vi "UHR-Fleezers Control (host) - Avogadro v1.vi"() -> ()   [LabVIEW 2014] (continued)
2.430581438642532, 2.430926786095764, 2.431356364635146, 2.4317856379894374, 2.4321182287057037, 2.432515152439944, 2.4328666951506044, 2.4333012482070333, 2.433380260628069, 2.4336372264778565, 2.433614551225319, 2.4335650502029416, 2.4334475234229562, 2.4333011261329975, 2.433007934812456, 2.432660908841205, 2.4323364970854775, 2.431945677053128, 2.4314603106784243, 2.4310055848872327, 2.4304504226813495, 2.429832483901481, 2.4295840632343437, 2.430289254432808, 2.430990173039951, 2.431600177007347, 2.4321969969786634, 2.4325847651600614, 2.432949278237247, 2.4332937711722127, 2.4336035035248855, 2.4338471633045415, 2.43411856440931, 2.4341327249977085, 2.434035584582046, 2.433841761528369, 2.4335344706564492, 2.4331067537461406, 2.4326152531510337, 2.4322612994781294, 2.4318525650807197, 2.4314216742454273, 2.431016113773001, 2.4305053865169173, 2.4301109347819363, 2.4296082033753423, 2.4291993469038955, 2.4287146214178863, 2.428318033387242, 2.427947843867298, 2.427710409863576, 2.4275749382000127, 2.427406750694291, 2.4272803430280403, 2.427055726798301, 2.4267129123813582, 2.426466566972866, 2.4265800653096097, 2.4264022339548923, 2.42636317026276, 2.4261367534409617, 2.4259769585253403, 2.4209620349742065, 2.420926541947684, 2.420983275856805, 2.4211451155125534, 2.4212160100100664, 2.421280648213139, 2.4213176976836435, 2.421396557512131, 2.4214452955717625, 2.4213891109958166, 2.4212491836298677, 2.42129685354167, 2.4214397106845302, 2.4216707358012615, 2.421910672322762, 2.422093997009182, 2.422323526718951, 2.422714682454901, 2.4230255439924244, 2.4235496993926793, 2.423987121189, 2.4243907895138364, 2.424590746787921, 2.4248405102694734, 2.4251454512161543, 2.425395336771748, 2.4256246223334412, 2.4256791894283816, 2.4256945402386467, 2.4256017639698415, 2.4255321207312166, 2.4253109836115545, 2.4250167851802042, 2.4246725974303374, 2.42415070039979, 2.423467665639209, 2.4229174169133496, 2.422391308328497, 2.4217404095583976, 2.4211572618793236, 2.4211068453016704, 2.421682821131013, 2.4222059999389587, 2.4226697897274634, 2.423094027527689, 2.4236765037995527, 2.4239891048921156, 2.424316080202641, 2.4245177770317685, 2.424673329874565, 2.424790337839895, 2.424709433271276, 2.4246918851283272, 2.424496749778738, 2.424243598742637, 2.4239404889065184, 2.423611957152008, 2.423288918729205, 2.4229048432874487, 2.422400921658983, 2.421536027100433, 2.421068910794393, 2.42072060304574, 2.4203089999084413, 2.420026642658768, 2.4196926480910648, 2.4193796807763888, 2.4190245674001263, 2.418800988799702, 2.418650532547986, 2.418678823206272, 2.4186175725577495, 2.4184317148350396, 2.418353709524823, 2.418170720542003, 2.418003967406226, 2.417792291024499, 2.4176316110721063, 2.4175349894711093, 2.4173629566331947, 2.417207373271886, 2.41730030213324, 2.4174544816431127, 2.4175632801293956, 2.417742790002129, 2.4180165410321286, 2.418110812707902, 2.4181535996581878, 2.418099612414924, 2.418115939817495, 2.417978545487829, 2.418120883816028, 2.4182416150395163, 2.4184165471358328, 2.418608569597455, 2.418898007141329, 2.419110782189396, 2.4194311349833684, 2.4197565538499073, 2.4202420422986477, 2.420669942320011, 2.4211170995208566, 2.4214806360057346, 2.4217368999297992, 2.422168858912926, 2.42250303659169, 2.4226787316507403, 2.422940610980556, 2.4229851069673676, 2.423065034943685, 2.423195989867848, 2.423032593768114, 2.4228180791650056, 2.422440992461923, 2.422032990508745, 2.421433820612196, 2.4209468062379784, 2.420461653492839, 2.4199261757255752, 2.4194091616565454, 2.419384411145355, 2.420076479384742, 2.420686025574504, 2.4213249000518786, 2.4217745902890058, 2.4222578508865595, 2.4227300332651676, 2.423039735099329, 2.4233286843470467, 2.423545365764331, 2.4236784875026656, 2.4237635120700705, 2.423771416364023, 2.4236595660267928, 2.423627063814199, 2.423647724845113, 2.4233858149967897, 2.4231237220374098, 2.4228541520432048, 2.4225346842860156, 2.4221234473708244, 2.42164976958525, 2.4213015839106395, 2.420928800317386, 2.420634083071378, 2.4201690725424907, 2.4198965422528707, 2.4196620685445707, 2.4194428540910047, 2.4193014923551144, 2.419234412671285, 2.419066042054504, 2.418075472273929, 2.4178200628681212, 2.417850154118468, 2.418008453627117, 2.4178781701101624, 2.4178394421216405, 2.417761833552041, 2.4177437055574154, 2.406593401898251, 2.4039209265419417, 2.4035707571642124, 2.4033807489242163, 2.4033286843470503, 2.403229651783802, 2.4031948301644883, 2.4032014831995547, 2.4031528366954533, 2.4030944242683163, 2.4030547196874847, 2.4031530808435244, 2.4033223975341, 2.40348313852351, 2.40359135715811, 2.403636158330024, 2.4037828302865623, 2.4041361735892806, 2.404406811731312, 2.4048561662648353, 2.405317697683637, 2.4055910214545078, 2.405806115909293, 2.406070070497755, 2.4062391125217393, 2.4064092226935587, 2.406426221503337, 2.4066071047090016, 2.4065373393963383, 2.4063661610766838, 2.4061467940305765, 2.4056369518112697, 2.405410107730332, 2.4051367839594686, 2.4046134830774855, 2.404083742789998, 2.4035795159764346, 2.4029824823755557, 2.402330027161473, 2.4015955992309306, 2.401533219397561, 2.4021967223120804, 2.402693655201877, 2.4032305063020662, 2.4036669820245944, 2.4041217383342954, 2.4044415417950957, 2.4046650288399882, 2.4048795434430934, 2.404969725638594, 2.4047648243659756, 2.4047524948881476, 2.404638966032896, 2.40437504196295, 2.40416742454298, 2.404013458662675, 2.4035543076876085, 2.4030866725669062, 2.40267934202093, 2.402205328531752, 2.401525803399758, 2.400994109927664, 2.4005073702200335, 2.4000125431073918, 2.399666432691425, 2.399542344431894, 2.3991321756645387, 2.398807275612653, 2.3985068819238817, 2.398275582140563, 2.398063081759082, 2.3979806817834977, 2.3978454847865187, 2.397760826441233, 2.397697225867489, 2.397577776421397, 2.3974082461012607, 2.3973235572374643, 2.3971585741752346, 2.3969482100894144, 2.399339609973449, 2.3996950895718228, 2.3997654957731838, 2.3997879573961587, 2.3999571214941846, 2.4000226142155188, 2.4000767235328184, 2.40004583880123, 2.4001323587755943, 2.4002205877864884, 2.400232245857111, 2.4004011047700407, 2.4005788750877337, 2.400797845393222, 2.401105594042782, 2.4016392406994806, 2.4019311502426213, 2.4022950529496114, 2.4027085787530114, 2.4032281868953476, 2.4037702871791677, 2.4041618091372414, 2.404428052613911, 2.404843684194461, 2.4051377300332626, 2.4055124362926077, 2.4056537064729686, 2.405908444471569, 2.4058568071535325, 2.4058369701223734, 2.4055328836939545, 2.4053381756035, 2.4050690023499244, 2.404632801293984, 2.4042121951963833, 2.4037009796441504, 2.4032916043580337, 2.4027538987395824, 2.4021463362529354, 2.401571764275031, 2.4014757225257117, 2.4020927152317855, 2.4026458632160357, 2.4031801507614308, 2.4036126590777247, 2.4041590929898926, 2.404629566331979, 2.4050496536149155, 2.4053699758903715, 2.405671163060388, 2.4060234687337823, 2.40607593005157, 2.4060553910946934, 2.4060759910885916, 2.4059835200048774, 2.405767418439276, 2.4055522934659828, 2.405272835474708, 2.4049551377910685, 2.4046062196722304, 2.403999328592787, 2.4035610522782016, 2.4032514419995685, 2.40294955290383, 2.4027128513443357, 2.402457594531081, 2.4022258674886334, 2.402022461622973, 2.4018425855281196, 2.401701437421794, 2.401658528397469, 2.4015787224951906, 2.401492141483804, 2.401444593646041, 2.4014353160191626, 2.401671651356542, 2.4017135837885633, 2.4018295846430813, 2.401837549974056, 2.4017239906002943, 2.424597918637651, 2.4246118350779726, 2.424565507980587, 2.42459965819269, 2.424594073305456, 2.4245285195471036, 2.4245402691732525, 2.4247233802301023, 2.424646931363866, 2.424751487777332, 2.4247339396343883, 2.424781212805563, 2.424835016937768, 2.4247366557817274, 2.4247208777123284, 2.424638264107179, 2.424499588000122, 2.4244687337870374, 2.424328531754507, 2.42422482985931, 2.4241373943296605, 2.424011902218693, 2.4236910306100627, 2.42360475478377, 2.4235302896206514, 2.4235555894650047, 2.4235575731681207, 2.4235125888851528, 2.42349827570421, 2.4234156010620382, 2.4232872707296917, 2.4231805169835416, 2.4231496932889733, 2.4230475478377596, 2.422977690969568, 2.4230106204412944, 2.4229536423841003, 2.4229382305368117, 2.422888180181274, 2.422950346385075, 2.4229270302438395, 2.4229190649128642, 2.4226663716544024, 2.4226755882442625, 2.422584673604535, 2.422560686056087, 2.4226352732932437, 2.4229356364635053, 2.4229169286171994, 2.4229865108188076, 2.424675008392584, 2.4252596514786156, 2.425283150730913, 2.4254429456465294, 2.4254956511123926, 2.425613177892387, 2.4259598071230144, 2.4260010681478272, 2.4260692770165075, 2.426234687337868, 2.4262993865779587, 2.4264269844660737, 2.426569872127441, 2.426780083620717, 2.4270130008850312, 2.427282967619854, 2.4273390301217663, 2.4276983855708405, 2.42808078249458, 2.4286301461836577, 2.4290816675313547, 2.4294141056550753, 2.4298842738120636, 2.430225898007133, 2.430553727835928, 2.4309037141026, 2.431134952848902, 2.431286141544846, 2.431253883480331, 2.431170751060514, 2.4310626850184627, 2.430942991424295, 2.430730918301947, 2.4304457228308918, 2.430165593432409, 2.4297568285164917, 2.4296153447065603, 2.4291805169835476, 2.428557847834706, 2.4280869472334916, 2.4281168858912854, 2.4287542954802084, 2.4295111545152106, 2.4301620838038196, 2.4307819147312806, 2.4313480025635523, 2.4315205542161324, 2.4318085879085625, 2.4321279335917176, 2.4323574938199934, 2.4325492721335404, 2.432612842188781, 2.432604907376317, 2.432455244605846, 2.432274117252107, 2.4319997863704295, 2.431997924741351, 2.431658742027037, 2.4312776573992108, 2.43085882137516, 2.4304665974913706, 2.429956236457407, 2.4296554155095036, 2.4292895596179056, 2.4290475478377633, 2.4287481612598, 2.428205755790881, 2.427885982848589, 2.4276909695730398, 2.4276541337320996, 2.4274905850398176, 2.4276107974486476, 2.4276034424878614, 2.4273903622547013, 2.427224982451853, 2.4271848200933808, 2.4269551988280877, 2.4267975402081343, 2.4267496261482577, 2.426536301767019, 2.402900875881221, 2.4031380657368633, 2.403752037110504, 2.4042728659932218, 2.4050129093295034, 2.4052575457014633, 2.4056152226325183, 2.405845484786517, 2.405950468459114, 2.405743491927848, 2.4051299783318587, 2.404316751609847, 2.404051820429085, 2.404275246436962, 2.404634113589891, 2.4047569811090383, 2.4051246070741885, 2.4055120090334725, 2.4058326670125365, 2.4063693044831678, 2.4067348857081807, 2.406775078585158, 2.4071752067628993, 2.407703695791494, 2.4078374584185243, 2.4081329691457833, 2.408269081698046, 2.408250526444283, 2.4082946256904774, 2.408282418286684, 2.4080811792351993, 2.4081080355235382, 2.4079442732016916, 2.407491012298956, 2.4070355235450283, 2.4066586809900175, 2.4060685750907864, 2.4054919278542384, 2.4049438764610716, 2.4042894070253564, 2.4041783196508693, 2.404856166264839, 2.405279549546793, 2.4057430646687172, 2.4062998138370912, 2.4066878872035886, 2.4067595446638355, 2.4071760307626544, 2.4073634144108387, 2.4075584582048983, 2.4076643879512893, 2.4077086703085353, 2.407621631519512, 2.4074461195715173, 2.4071774346140895, 2.4067588427381175, 2.4066013977477314, 2.406143955809193, 2.405616870632034, 2.4051503952146938, 2.4046809900204456, 2.4041257972960577, 2.4037431867427563, 2.403418012024289, 2.4030837122714876, 2.402824457533492, 2.4025822931608016, 2.4023588061159042, 2.402216620380259, 2.4021348612933697, 2.401934965056304, 2.401611224707785, 2.4014654683065273, 2.401353160191649, 2.40129486983855, 2.4013071077608505, 2.4011179235206104, 2.4010649128696504, 2.400908413953057, 2.400771691030605, 2.4020871303445483, 2.4011822260200764, 2.4007248451185617, 2.4004102298043732, 2.3998872951445063, 2.399638630329293, 2.3994718771935144, 2.399311044648575, 2.39913538010803, 2.399068422498242, 2.398960966826375, 2.3986503494369287, 2.3986418958098024, 2.398676351207001, 2.3988180181279932, 2.398978362376777, 2.3994265877254564, 2.3998741111484096, 2.4001463972899555, 2.4005340433973146, 2.4009977416302934, 2.401073030793167, 2.4014315622424993, 2.401741813409832, 2.40197305215613, 2.4023876766258674, 2.4026499526963048, 2.402819330423898, 2.402831354716631, 2.4027815790276805, 2.402703329569381, 2.4028177129428956, 2.4025652333140015, 2.402136692403945, 2.40164436780907, 2.400992217780078, 2.4004347361674796, 2.4000155034028174, 2.3995320902127117, 2.3990206610309106, 2.3991094698934887, 2.3998409070100983, 2.400514847254854, 2.4011603442487814, 2.401726035340429, 2.4021230506302067, 2.402113071077605, 2.4025136875514983, 2.4026888027588678, 2.4028879665517118, 2.4027249366740917, 2.4025446333201073, 2.402652150028987, 2.402734397412022, 2.402406781212803, 2.402132328257089, 2.4022540971098962, 2.4020598773155912, 2.40171459089938, 2.401353556932273, 2.4009453413495225, 2.400347270119321, 2.400007446516312, 2.399501022370065, 2.3991158482619657, 2.39877190466017, 2.398409833063749, 2.3981063264870137, 2.3978381298257374, 2.397473036896876, 2.3972162541581454, 2.396722952970971, 2.3964001892147513, 2.3962673421430067, 2.3961395306253186, 2.396097903378391, 2.39589822077089, 2.3957543565172243, 2.3955935239722863, 2.3953248084963525, 2.3711730704672336, 2.3691772515030287, 2.368657460249641, 2.368525070955532, 2.368504135258033, 2.3685816522720984, 2.369277321695607, 2.369537125766776, 2.3694836878566834, 2.3696178167058295, 2.3696047242652627, 2.3696505325479884, 2.369786339915157, 2.369958159123507, 2.3701187780388797, 2.3703828547013766, 2.3703139744254886, 2.3705926999725313, 2.3709521469771375, 2.371376079592269, 2.371703726310003, 2.372084261604661, 2.372402600177005, 2.3726291390728416, 2.372854182561725, 2.3730838648640367, 2.3734214300973506, 2.3735248878444755, 2.373402447584457, 2.3732737815485083, 2.373095217749563, 2.3729121982482355, 2.3726266060365604, 2.372233710745564, 2.371795739616075, 2.371224280526134, 2.370653157139803, 2.3700431836909024, 2.369352122562329, 2.3686639912106693, 2.368520035401466, 2.3687518234809373, 2.3692865382854666, 2.369742362743001, 2.3701869258705393, 2.370600848414558, 2.370890102847375, 2.371232123783071, 2.3714059266945355, 2.371503616443369, 2.3714757835627265, 2.371450148014769, 2.371331064790795, 2.371147282326728, 2.3709205603198336, 2.370594347972041, 2.3701680654316837, 2.369824732200076, 2.369418927579573, 2.369010559404277, 2.368637379070405, 2.3684136173589247, 2.368100344859156, 2.367791741691333, 2.367505630664996, 2.36728153324991, 2.3670190130314013, 2.3668691671498707, 2.366697531052578, 2.36665858943449, 2.3665348979155816, 2.3662927030243854, 2.366204962309637, 2.366202612384408, 2.3661817987609473, 2.3661056550798043, 2.3660763878292177, 2.366077394940028, 2.3660827051606765, 2.36617389446699] caption="Most Recent Time Trace"
  out "Values":dbl[](array[numeric])=[-0.06760925671124465, 0.04910653407946759, 4.445727607043673, -0.09151692288622436, 0.04947272910700923, 3.2662948698385565, -0.09383489136567569, 3.086667088839382, -0.1922671172735984, 2.235330652790918, -0.05378544658904728, -0.006441883611510604, 2.422861781670583]
  out "All Signals":waveform(dbl)[](graph)=[{"t0"=timestamp(302.5999999999914 s since 1904-01-01), "dt"=0.15, "Y"=[0.0], "attributes"=variant("NI_ChannelName"=variant(string "APD 1"))}, {"t0"=timestamp(302.5999999999914 s since 1904-01-01), "dt"=0.15, "Y"=[0.0], "attributes"=variant("NI_ChannelName"=variant(string "APD 2"))}, {"t0"=timestamp(302.5999999999914 s since 1904-01-01), "dt"=0.15, "Y"=[0.0], "attributes"=variant("NI_ChannelName"=variant(string "APD 3"))}, {"t0"=timestamp(302.5999999999914 s since 1904-01-01), "dt"=0.1, "Y"=[-0.06757372680085764, -0.06764478662163165], "attributes"=variant("NI_ChannelName"=variant(string "T1 Y"))}, {"t0"=timestamp(302.5999999999914 s since 1904-01-01), "dt"=0.1, "Y"=[0.049145059705078195, 0.0490680084538571], "attributes"=variant("NI_ChannelName"=variant(string "T1 X"))}, {"t0"=timestamp(302.5999999999914 s since 1904-01-01), "dt"=0.1, "Y"=[4.445783654286312, 4.445671559801015], "attributes"=variant("NI_ChannelName"=variant(string "T1 Sum"))}, {"t0"=timestamp(302.5999999999914 s since 1904-01-01), "dt"=0.1, "Y"=[-0.09151746422952804, -0.09151638154292077], "attributes"=variant("NI_ChannelName"=variant(string "T2 Y"))}, {"t0"=timestamp(302.5999999999914 s since 1904-01-01), "dt"=0.1, "Y"=[0.04952704956149684, 0.04941840865252152], "attributes"=variant("NI_ChannelName"=variant(string "T2 X"))}, {"t0"=timestamp(302.5999999999914 s since 1904-01-01), "dt"=0.1, "Y"=[3.266107669301433, 3.2664820703756816], "attributes"=variant("NI_ChannelName"=variant(string "T2 Sum"))}, {"t0"=timestamp(302.5999999999914 s since 1904-01-01), "dt"=0.1, "Y"=[-0.09387435236185547, -0.0937954303694959], "attributes"=variant("NI_ChannelName"=variant(string "T1 FB X"))}, {"t0"=timestamp(302.5999999999914 s since 1904-01-01), "dt"=0.1, "Y"=[3.0867849971007453, 3.0865491805780243], "attributes"=variant("NI_ChannelName"=variant(string "T1 FB Sum"))}, {"t0"=timestamp(302.5999999999914 s since 1904-01-01), "dt"=0.1, "Y"=[-0.192305278199375, -0.19222895634782178], "attributes"=variant("NI_ChannelName"=variant(string "T2 FB X"))}, {"t0"=timestamp(302.5999999999914 s since 1904-01-01), "dt"=0.1, "Y"=[2.2353390301217684, 2.235322275460067], "attributes"=variant("NI_ChannelName"=variant(string "T2 FB Sum"))}, {"t0"=timestamp(302.5999999999914 s since 1904-01-01), "dt"=0.1, "Y"=[-0.053826675533845625, -0.05374421764424899], "attributes"=variant("NI_ChannelName"=variant(string "T3 Y/ PSD Y"))}, {"t0"=timestamp(302.5999999999914 s since 1904-01-01), "dt"=0.1, "Y"=[-0.006535476968530134, -0.006348290254491073], "attributes"=variant("NI_ChannelName"=variant(string "T3 X / PSD X"))}, {"t0"=timestamp(302.5999999999914 s since 1904-01-01), "dt"=0.1, "Y"=[2.422819391460915, 2.422904171880237], "attributes"=variant("NI_ChannelName"=variant(string "T3 Sum / PSD sum"))}]
  in  "Signals to Plot":i32(listbox)=18
  out "Trap Disp. Freq. (Hz)":dbl=10.0 caption="Freq. (Hz)" format="%#_6p"
  out "Display Period (s)":dbl=0.1 caption="Period (s)" format="%#_6p"
  in  "Trap Disp. Downsample":dbl=10000.0 caption="Downsample" max=20000.0
  in  "APD Disp. Scale":dbl=0.1 caption="Scale (Divide,\nfor above plot only)"
  in  "APD Disp. Downsample":dbl=150.0 caption="Integrate" max=200.0
  out "APD Display Freq. (Hz)":dbl=6.666666666666667 caption="Freq. (Hz)"
  out "APD Display Period (s)":dbl=0.15 caption="Period (s)"
  out "FFT 1":cluster{"f0":dbl, "df":dbl, "magnitude":dbl[]}[](graph)=[{"f0"=0.0, "df"=3.3333333333333335, "magnitude"=array[10000 elements]}, {"f0"=0.0, "df"=3.3333333333333335, "magnitude"=array[10000 elements]}]
  out "FFT 2":cluster{"f0":dbl, "df":dbl, "magnitude":dbl[]}[](graph)
  in  "FFT 1 Choice 1":u16(ring) items=["T1 Y", "T1 X", "T1 Sum", "T2 Y", "T2 X", "T2 Sum", "T1 FB X", "T1 FB Sum", "T2 FB X", "T2 FB Sum", "PSD Y", "PSD X", "PSD Y Sum", "none"]
  in  "FFT 2 Choice 1":u16(ring)=13 items=["T1 Y", "T1 X", "T1 Sum", "T2 Y", "T2 X", "T2 Sum", "T1 FB X", "T1 FB Sum", "T2 FB X", "T2 FB Sum", "PSD Y", "PSD X", "PSD Y Sum", "none"]
  in  "FFT 1 Choice 2":u16(ring)=1 items=["T1 Y", "T1 X", "T1 Sum", "T2 Y", "T2 X", "T2 Sum", "T1 FB X", "T1 FB Sum", "T2 FB X", "T2 FB Sum", "PSD Y", "PSD X", "PSD Y Sum", "none"]
  in  "FFT 2 Choice 2":u16(ring)=13 items=["T1 Y", "T1 X", "T1 Sum", "T2 Y", "T2 X", "T2 Sum", "T1 FB X", "T1 FB Sum", "T2 FB X", "T2 FB Sum", "PSD Y", "PSD X", "PSD Y Sum", "none"]
  in  "Compute FFT":bool
  in  "Reset FFT":bool
  in  "# Spectra to Ave.":dbl=25.0
  out "Ave. Time (s)":dbl=7.5
  out "1 Channel":waveform(dbl)(graph)={"t0"=timestamp(0 s since 1904-01-01), "dt"=1e-05, "Y"=array[20000 elements], "attributes"=variant("NI_ChannelName"=variant(string "T1 X"))}
  out "Slow mean":dbl=0.04910653407946759 format="%0.2f"
  in  "Slow mean N ave.":dbl=1.0 min=1.0 step=1.0
  out "Mean Intensity":dbl=0.049106534079467676
  out "Sigma":dbl=0.00020183735235839546
  out "Sigma/Mean":dbl=0.004110193401793903
  in  "Subtract mean":bool
  in  "High Res. Display":u16(ring)=1 items=["T1 Y", "T1 X", "T1 Sum", "T2 Y", "T2 X", "T2 Sum", "T1 FB X", "T1 FB Sum", "T2 FB X", "T2 FB Sum", "PSD Y", "PSD X", "PSD Y Sum"]
  out "Positions \nand displacements":cluster{"X":dbl[], "Y":dbl[]}[](graph)=[{"X"=[3248.000000000121, 3248.000000000121, 3248.000000000121, 3248.000000000121, 3248.000000000121, 3248.000000000121, 3248.000000000121, 3248.000000000121, 3248.000000000121, 3248.000000000121, 3248.000000000121, 3248.000000000121, 3248.000000000121, 3248.000000000121, 3248.000000000121, 3248.000000000121, 3248.000000000121, 3248.000000000121, 3248.000000000121, 3248.000000000121], "Y"=[0.0, 0.0, 0.0, 0.0, 0.0, 0.0, 0.0, 0.0, 0.0, 0.0, 0.0, 0.0, 0.0, 0.0, 0.0, 0.0, 0.0, 0.0, 0.0, 0.0]}, {"X"=[6090.0, 6090.0, 6090.0, 6090.0, 6090.0, 6090.0, 6090.0, 6090.0, 6090.0, 6090.0, 6090.0, 6090.0, 6090.0, 6090.0, 6090.0, 6090.0, 6090.0, 6090.0, 6090.0, 6090.0], "Y"=[0.0, 0.0, 0.0, 0.0, 0.0, 0.0, 0.0, 0.0, 0.0, 0.0, 0.0, 0.0, 0.0, 0.0, 0.0, 0.0, 0.0, 0.0, 0.0, 0.0]}, {"X"=[2307.4241248817407, 2307.4241248817407, 2307.4241248817407, 2307.4241248817407, 2307.4241248817407, 2307.4241248817407, 2307.4241248817407, 2307.4241248817407, 2307.4241248817407, 2307.4241248817407, 2307.4241248817407, 2307.4241248817407, 2307.4241248817407, 2307.4241248817407, 2307.4241248817407, 2307.4241248817407, 2307.4241248817407, 2307.4241248817407, 2307.4241248817407, 2307.4241248817407], "Y"=[-2608.415338602863, -2608.415338602863, -2608.415338602863, -2608.415338602863, -2608.415338602863, -2608.415338602863, -2608.415338602863, -2608.415338602863, -2608.415338602863, -2608.415338602863, -2608.415338602863, -2608.415338602863, -2608.415338602863, -2608.415338602863, -2608.415338602863, -2608.415338602863, -2608.415338602863, -2608.415338602863, -2608.415338602863, -2608.415338602863]}]
  in  "Tab Control":T8(tab)=enum."Trap Control (RF)"
  in  "T3 calibration":T9={"alpha_x (nm/V)"=4469.800261295657, "offset_x (mV)"=-6.864397522963529, "kappa_x (pN/nm)"=1.1601247758607456, "alpha_y (nm/V)"=3755.02211097385, "kappa_y (pN/nm)"=0.9477281505140224, "offset_y (mV)"=-50.86424092307882} {"offset_y (mV)" format="%#_2g"; "kappa_y (pN/nm)" min=0.0 step=0.001 format="%#_2g"; "alpha_y (nm/V)" step=10.0 format="%#_3g"; "kappa_x (pN/nm)" min=0.0 step=0.001 format="%#_2g"; "offset_x (mV)" format="%#_2g"; "alpha_x (nm/V)" step=10.0 format="%#_3g"}
  in  "T2 calibration":T9={"alpha_x (nm/V)"=15035.499369253672, "offset_x (mV)"=53.40070864855844, "kappa_x (pN/nm)"=0.8476828823436685, "alpha_y (nm/V)"=9629.48354749487, "kappa_y (pN/nm)"=1.7582670013917883, "offset_y (mV)"=-92.95284747435186} {"offset_y (mV)" format="%#_2g"; "kappa_y (pN/nm)" min=0.0 step=0.001 format="%#_2g"; "alpha_y (nm/V)" step=10.0 format="%#_3g"; "kappa_x (pN/nm)" min=0.0 step=0.001 format="%#_2g"; "offset_x (mV)" format="%#_2g"; "alpha_x (nm/V)" step=10.0 format="%#_3g"}
  in  "Visa resource for valves":refnum<visa-resource-name>="COM10"
  in  "Cursor control":cluster{"X":bool, "Y":bool}={"X"=TRUE, "Y"=TRUE}
  in  "Trap 3 (ON/OFF)":bool=TRUE
  in  "Maximum Delta\n(MHz)":dbl=30.0
  in  "T3 Y (V)":dbl min=0.0 max=10.0 step=1.0 format="%#_6f"
  in  "T3 X (V)":dbl=10.0 min=0.0 max=10.0 step=1.0 format="%#_6f"
  in  "Shunt 1":bool caption="Inject Pump 3"
  in  "manual raster set":u16(ring) items=["offset", "user-defined", "basepaire step", "user-defined 2", "user-defined 3", "user-defined 4"]
  in  "move Con X?":bool
  in  "Symmetric?":bool
  out "Laser Intensity Low (bugs to fix)":bool
  out "Good freq?":bool=TRUE
  in  "T1 calibration":T9={"alpha_x (nm/V)"=17437.401805668047, "offset_x (mV)"=52.75299645671799, "kappa_x (pN/nm)"=0.7040228768485087, "alpha_y (nm/V)"=9389.781729819388, "kappa_y (pN/nm)"=1.842787790887783, "offset_y (mV)"=-70.0338515440209} {"offset_y (mV)" format="%#_2g"; "kappa_y (pN/nm)" min=0.0 step=0.001 format="%#_2g"; "alpha_y (nm/V)" step=10.0 format="%#_3g"; "kappa_x (pN/nm)" min=0.0 step=0.001 format="%#_2g"; "offset_x (mV)" format="%#_2g"; "alpha_x (nm/V)" step=10.0 format="%#_3g"}
  in  "Blue FB Setpoint (mV)":dbl=90.0
  in  "Blue Laser ON":bool
  in  "11":bool
  out "Stage Moving":bool
  in  "Read Cal":bool
  in  "Speed (nm/s)":dbl=100.0
  in  "Furthest Withdraw (MHz)":dbl=15.0
  in  "Round T1 X":bool caption="Round"
  in  "Cal sets to save":u32=25 min=1 step=1
  in  "Trap 2 (ON/OFF)":bool=TRUE
  in  "Trap 1 (ON/OFF)":bool=TRUE
  in  "Save Calibration":bool
  out "Manipulating Trap":bool
  out "Buffer Status":dbl(slide)=5.172413793103448e-06 scale=0.0..1.0
  out "Overflow (data lost)":bool
  in  "Reset":bool
  out "Data Rate (Hz)":dbl=100000.0 caption="Trap Data Rate (Hz)" format="%#_3p"
  out "Data Period (s)":dbl=1e-05 caption="Trap Data Period (s)" format="%#_6p"
  in  "BD 1 Frequency 1 (MHz)":dbl=76.0 caption="T1 X (MHz)" min=60.0 max=90.0 step=1.0 format="%#_6p"
  in  "BD 1 Frequency 2 (MHz)":dbl=90.0 caption="T2 X (MHz)" min=60.0 max=90.0 step=1.0 format="%#_6p"
  in  "Round T2 X":bool caption="Round"
  in  "Trap Raster Scan":bool
  out "Raster Scanning...":bool
  in  "Trap Delta (MHz)":dbl=14.0
  in  "Setpoints (V)":cluster{"Set 1":dbl, "Set 2":dbl}={"Set 1"=2.0, "Set 2"=2.0}
  in  "Fish for Tether":bool
  in  "Red FB Setpoint (mV)":dbl=100.0
  in  "Confocal Linescan":bool
  in  "Confocal Image":bool
  in  "Green Laser ON":bool
  in  "AO1":dbl(slide)=0.7905362102114931 caption="Confocal Y (V)" min=0.0 max=10.0 step=0.01 scale=0.0..10.0 scale format="%_1f"
  in  "AO2":dbl(slide)=4.726554155095066 caption="Confocal X (V)" min=0.0 max=10.0 step=0.01 scale=0.0..10.0 scale format="%_1f"
  in  "Green FB Setpoint (mV)":dbl=200.0
  in  "Red Laser ON":bool
  in  "Active Cal":bool
  out "A cal freq (Hz)":dbl=500.0 caption="Freq. (Hz)"
  in  "Laser interlacing mode":enum32{"Laser ON", "Laser OFF", "Interlace"}(radio)=enum."Interlace" caption="Laser interlacing mode (all lasers)"
  in  "Green Intensity % (FB OFF)":dbl=7.0 min=0.0 max=100.0 step=1.0
  in  "Shunt 2":bool caption="Inject Pump 3"
  out "Piezo trap cursor control":cluster{"X":dbl, "Y":dbl}[](graph)
  in  "Scan trap 3 or Fl?":bool=TRUE
  in  "Position Label 6":string="0 position (don't change)" caption="6"
  in  "Move to Position 6":bool
  in  "Set Position 6":bool
  in  "Position Label 5":string="central flow spot (UvrD)" caption="5"
  in  "Move to Position":bool
  in  "Position":dbl=1.0 min=1.0 max=10.0 step=1.0
  in  "Set Position":bool
  in  "Saved Stage Positions":dbl[][](array[numeric])=[[1.0, 1.13999, 0.68071, -0.08115], [2.0, -0.93838, -0.06724, -0.08115], [3.0, -1.0896, 0.54048, -0.08115], [4.0, 0.0, 0.0, 0.0], [5.0, 0.64634, 0.24639, 0.00962], [6.0, 0.0, 0.0, 0.0], [7.0, 0.0, 0.0, 0.0], [8.0, 0.0, 0.0, 0.0], [9.0, 0.0, 0.0, 0.0], [10.0, 0.0, 0.0, 0.0]]
  in  "Move to Position 5":bool
  in  "Position 1 Label":string="Position 1 (lower left)" caption="1"
  in  "Set Position 1":bool
  in  "Set Position 2":bool
  in  "Set Position 3":bool
  in  "Set Position 4":bool
  in  "Move to Position 3":bool
  in  "Move to Position 4":bool
  in  "Move to Position 2":bool
  in  "Move to Position 1":bool
  in  "Position 2 Label":string="Position 2 (upper right)" caption="2"
  in  "Position 3 Label":string="Position 3 (lower right)" caption="3"
  in  "Position 4 Label":string="Experiment position" caption="4"
  in  "Set Position 5":bool
  out "Stage Control Serial Error":errorcluster
  in  "y nudge increment (um":dbl=0.5
  in  "-y":bool
  in  "+y":bool
  in  "x nudge increment (um)":dbl=0.5
  in  "-x":bool
  in  "+x":bool
  in  "-z":bool
  in  "+z":bool
  in  "z nudge increment (um)":dbl=0.5
  in  "Pressure Pump Voltage (+/-10V)":dbl
  in  "Use Harvard pumps\nfor beads (else Chemyx)":bool=TRUE
  in  "Tab Control 9":enum32{"Harvard Pumps", "Chemyx Pumps"}(tab)
  in  "Display On P3":bool caption="Display On"
  in  "Normal Flow Rate (ul/h) P3":dbl=800.0 caption="Normal Flow Rate (ul/h)"
  out "Flushing P3":bool caption="Flushing"
  in  "Retract Vol 1 (uL)":dbl=250.0 caption="Volume (uL)"
  in  "Retract Vol 3 (uL)":dbl=250.0 caption="Volume (uL)"
  in  "Retract Rate (uL/m)":dbl=2000.0
  in  "Retract Pump 1":bool
  in  "Retract Pump 3":bool
  in  "Stop Flow":bool
  in  "Start Flow":bool
  in  "Flush Sample":bool
  in  "Volume (uL)":dbl=100.0
  in  "Flush rate (uL/m)":dbl=100.0
  in  "Flow rate (uL/h)":dbl=100.0
  in  "Clear Volume":bool caption="Clear Infused Volume"
  in  "Flush Pump 3":bool
  in  "Volume (uL) P3":dbl=150.0 caption="Volume (uL)"
  in  "Flush rate (uL/m) P3":dbl=100.0 caption="Rate (uL/m)"
  out "Flushing P1":bool caption="Flushing"
  in  "Volume (uL) P1":dbl=100.0 caption="Volume (uL)"
  in  "Flush rate (uL/m) P1":dbl=100.0 caption="Rate (uL/m)"
  in  "Normal Flow Rate (ul/h) P1":dbl=600.0 caption="Normal Flow Rate (ul/h)"
  in  "Flush Pump 1":bool
  in  "Clear Volume P3":bool caption="Clear Infused Volume"
  in  "Clear Volume P1":bool caption="Clear Infused Volume"
  in  "Display On P1":bool caption="Display On"
  in  "All Pump Parameters":T10={"Pump 1"={"Diameter (mm)"=4.61, "Units"=4.0, "Volume"=100.0, "Rate"=25.0}, "Pump 2"={"Diameter (mm)"=4.61, "Units"=3.0, "Volume"=0.0, "Rate"=0.0}, "Pump 3"={"Diameter (mm)"=4.61, "Units"=4.0, "Volume"=100.0, "Rate"=800.0}}
  in  "Total Volume\nFlushed (uL)":dbl
  in  "Inject Pump 2":bool caption="Inject Pump 2\n(Flush Center)"
  in  "Flush Center Ch Rate (ul/m)":dbl=100.0
  in  "Flush Center Ch Volume (uL)":dbl=15.0
  in  "Pump pause delay (ms)":u32
  in  "Pump write delay (ms)":dbl=300.0
  in  "Ch 3 Inject Rate (ul/h)":dbl=800.0
  in  "Ch 3 Inject Volume (uL)":dbl=100.0
  in  "Ch 1 Inject Volume (uL)":dbl=100.0
  in  "Ch 1 Inject Rate (ul/h)":dbl=25.0
  out "Pump 1 cont disp":string="Right: DNA beads "
  out "Pump 3 cont disp":string="Left: ADig beads"
  in  "Read Harvard":bool
  out "read buffer":string
  out "Serial Settings:Number of Bytes at Serial Port":u32
  in  "write buffer":string
  in  "Tab Control 2":T11(tab)=enum."AOD Raster Scan"
  in  "Update all trap values":bool
  out "Total Counts (ticks)":u16=400
  in  "Trap ON/OFF X or Y Amp?":bool=TRUE
  in  "Oscillate Set 1":bool
  in  "Trap 1 ON":bool=TRUE
  in  "Number Interlace Sets":u8=2 min=1 max=3
  in  "DIO count 3 (ticks)":u16=200
  in  "DIO count 2 (ticks)":u16=200
  in  "DIO count 1 (ticks)":u16=200
  in  "BD 2 Amplitude 3 (%)":dbl min=0.0 max=45.0 step=1.0
  in  "BD 2 Amplitude 2 (%)":dbl min=0.0 max=45.0 step=1.0
  in  "BD 2 Amplitude 1 (%)":dbl min=0.0 max=45.0 step=1.0
  in  "BD 1 Amplitude 3 (%)":dbl min=0.0 max=50.0 step=1.0
  in  "BD 1 Amplitude 2 (%)":dbl=44.0 min=0.0 max=50.0 step=1.0
  in  "BD 1 Amplitude 1 (%)":dbl=45.0 min=0.0 max=50.0 step=1.0
  in  "BD 2 Frequency 3 (MHz)":dbl=26.0 min=0.0 max=40.0 step=0.1 format="%#_6p"
  in  "BD 1 Frequency 3 (MHz)":dbl=70.0 min=60.0 max=90.0 step=1.0 format="%#_6p"
  in  "BD 2 Frequency 2 (MHz)":dbl=26.0 min=0.0 max=40.0 step=0.1 format="%#_6p"
  in  "BD 2 Frequency 1 (MHz)":dbl=26.0 min=0.0 max=40.0 step=0.1 format="%#_6p"
  in  "Not-Interlacing Set":enum32{"Set 1", "Set 2", "Set 3"}(radio)
  in  "Interlace":bool=TRUE
  in  "Trap 2 ON":bool=TRUE
  in  "Trap 3 ON":bool
  in  "Scan axis 2":bool=TRUE
  in  "Osc. amp. (MHz)":dbl=2.0
  out "Coords":T12
  in  "Manipulation Scaling":cluster{"Horizontal":dbl, "Vertical":dbl}={"Horizontal"=0.075, "Vertical"=0.01}
  in  "Freq or Amp switch first":bool=TRUE
  in  "Swap F1 and F2":bool
  in  "Freq switch delay":u16
  in  "Amp switch delay":u16=7
  in  "BD 1 Delay (ticks)":u8
  in  "BD 2 Delay (Ticks)":u8
  in  "Next trap write delay (ticks)":u8
  in  "XY phase ext loop method":bool
  in  "Amp switch delay 2":u8=5
  in  "BD 2 Delay (Ticks) 2":u8
  in  "BD 1 Delay (ticks) 2":u8
  in  "MCL Step Increment (V_int)":dbl=3.0
  out "Time to Finish All (min)":dbl=0.5333333333333333 format="%#_2p"
  in  "Scan Speed (nm/s)":dbl=500.0
  in  "Scan Range (nm)":dbl=2000.0
  in  "Step Size (nm)":dbl=1.0
  in  "MCL/AOM Scale Tweak":dbl=1.0
  in  "MCL Step Position Ratio":dbl=0.5
  in  "Move MCL Also?":bool=TRUE
  out "Final sep (nm)":dbl=2123.8226600985217
  out "Initial sep (nm)":dbl=912.0
  out "Save index":dbl=27.0
  out "Final delta (MHz)":dbl=23.85221674876847
  out "Initial delta (MHz)":dbl=14.0
  out "Final freq. (MHz)":dbl=66.14778325123153
  out "Initial freq. (MHz)":dbl=76.0
  in  "Saved AOD Raster Scan Parameter Sets":T13(array[cluster])=[{"Scan Range AOD (nm) 2"=2000.0, "Step Size AOD (nm) 2"=1.0, "Scan Speed AOD (nm/s) 2"=500.0, "Number of scans (AOD) 2"=1, "Label"="offset curve"}, {"Scan Range AOD (nm) 2"=450.0, "Step Size AOD (nm) 2"=1.0, "Scan Speed AOD (nm/s) 2"=100.0, "Number of scans (AOD) 2"=1, "Label"="hp raster check"}, {"Scan Range AOD (nm) 2"=6.8, "Step Size AOD (nm) 2"=0.34, "Scan Speed AOD (nm/s) 2"=0.34, "Number of scans (AOD) 2"=1, "Label"="3.4 kbp - 1 bp steps"}, {"Scan Range AOD (nm) 2"=215.0, "Step Size AOD (nm) 2"=1.0, "Scan Speed AOD (nm/s) 2"=100.0, "Number of scans (AOD) 2"=3, "Label"="dt14 1 14 MHz start"}, {"Scan Range AOD (nm) 2"=450.0, "Step Size AOD (nm) 2"=1.0, "Scan Speed AOD (nm/s) 2"=100.0, "Number of scans (AOD) 2"=1, "Label"="dt14 2 small beads"}, {"Scan Range AOD (nm) 2"=300.0, "Step Size AOD (nm) 2"=1.0, "Scan Speed AOD (nm/s) 2"=100.0, "Number of scans (AOD) 2"=1, "Label"="Oligo"}]
  in  "Load parameters":bool
  out "Scan Range (MHz)":dbl=-9.852216748768473
  in  "Restart DMA? (AOD)":bool=TRUE caption="Restart DMA?"
  out "Incr. int (AOD)":i64=-4701660970
  out "Time/Scan (s) (AOD)":dbl=4.0 format="%#_2p"
  out "Data points/scans":dbl=3200000.0
  out "Data points/scan (f/b)":dbl=800000.0
  in  "Save scans":bool=TRUE
  out "AOD Scan I":u64=5 caption="Scan I"
  in  "Continuous AOD Scanning":bool caption="Continuous Scanning"
  in  "Abort AOD Scan":bool caption="Abort Scan"
  in  "Scan BD":bool=TRUE
  out "Cycles/step (AOD)":u64=200 format="%.3p"
  in  "Number of F/B Scans (AOD)":u16=4 min=1
  out "Scan steps (AOD)":u64=2000
  out "Scan Increment (MHz)":dbl=-0.004928572660714594
  out "AOD Scanning":bool caption="Scanning"
  in  "Start AOD Scan":bool caption="Start Scan"
  out "N sets should be saved":dbl=160.0
  out "Progress 2":u16(slide) caption="Progress" scale=0.0..100.0
  in  "Abort save 2":bool caption="Abort save"
  in  "Trap 1 Bead Size (nm)":dbl=810.0
  in  "Trap 2 Bead Size (nm)":dbl=810.0
  out "MCL Count":dbl=12036.500137333293
  in  "Feedback Auto-Off threshold":dbl=9.5
  in  "Trap intensity output range":cluster{"Normal High":i16, "Normal Low":i16}={"Normal High"=3000, "Normal Low"=0}
  in  "All FB On/Off":bool
  in  "AI2 to Setpoint":cluster{"Set 1":bool, "Set 2":bool}
  out "AI2 (V)":cluster{"Set 1":dbl, "Set 2":dbl}={"Set 1"=3.0826746421704767, "Set 2"=2.237311929685354}
  in  "Reset Feedback":cluster{"Set 1":bool, "Set 2":bool}
  in  "Trap Intensity PID Gains":T14={"proportional gain (Kc)"=10, "integral gain (Kc*Ts/Ti)"=5, "derivative gain (Kc*Td/Ts)"=0}
  in  "Feedback On/Off":cluster{"Set 1":bool, "Set 2":bool}={"Set 1"=TRUE, "Set 2"=TRUE}
  out "Actual Setpoint":fxp<+/-,16,1> format="%.16g"
  in  "Dynamic Force FB (ronen)":bool=TRUE
  in  "Remove Unwinding Offset":bool
  in  "Set Reading to\nSetpoint":bool
  out "Trap X (AI1)":T15={"Trap 1"=-0.04925537109375, "Trap 2"=-0.04937744140625}